vi "Dresden R2R Sputter 03.02.2018 IY24.vi"() -> ()   [LabVIEW 2009] (continued)
        n4396 = Boolean Array To Number(Boolean array=w6390) -> (number=w6389:u32)
        n4397 = Boolean Array To Number(Boolean array=w6370) -> (number=w6369:u32)
        n4398 = Boolean Array To Number(Boolean array=w6382) -> (number=w6383:u32)
        n4399 = Boolean Array To Number(Boolean array=w6357) -> (number=w6358:u32)
        n4400 = Boolean Array To Number(Boolean array=w6346) -> (number=w6345:u32)
        n4401 = Mantissa & Exponent(0:w6389) -> (2:w6388:dbl)  [unwired: 1 out]
        n4402 = Mantissa & Exponent(0:w6369) -> (2:w6366:dbl)  [unwired: 1 out]
        n4403 = Mantissa & Exponent(0:w6383) -> (2:w6378:dbl)  [unwired: 1 out]
        n4404 = Mantissa & Exponent(0:w6358) -> (2:w6361:dbl)  [unwired: 1 out]
        n4405 = Mantissa & Exponent(0:w6345) -> (2:w6344:dbl)  [unwired: 1 out]
        n4406 = case shown="1" w6388 {
          tunnel: [u32[][] [] ("data (RGB format)") w6403 w6404 w6405] -> w6387
          tunnel: w6386 -> [_ w6403 _ _]
          tunnel: w6384 -> [_ _ w6404 _]
          tunnel: w6333 -> [_ _ _ w6405]
          frame #0 {
            (unwired) cluster{"x":i16, "y":i16} {"x"=0, "y"=0} ("top left point(0, 0)")
          }
          frame #1 {
          }
          frame #2 {
          }
          frame #3 {
          }
        }
        n4407 = case shown="1" w6378 {
          tunnel: [u32[][] [] ("data (RGB format)") w6400 w6401] -> w6380
          tunnel: w6379 -> [_ w6400 _]
          tunnel: w6374 -> [_ _ w6401]
          frame #0 {
          }
          frame #1 {
          }
          frame #2 {
          }
        }
        n4408 = case shown="0, Default" w6366 {
          tunnel: w6365 -> [_ w6398]
          tunnel: [u32[][] [] ("data (RGB format)") w6398] -> w6363
          frame #0 {
          }
          frame #1 {
          }
        }
        n4409 = case shown="2" w6361 {
          tunnel: w6356 -> [_ w6395 _]
          tunnel: [u32[][] [] ("data (RGB format)") w6395 w6396] -> w6362
          tunnel: w6355 -> [_ _ w6396]
          frame #0 {
          }
          frame #1 {
          }
          frame #2 {
          }
        }
        n4410 = case shown="0, Default" w6344 {
          tunnel: w6342 -> [_ w6392 _]
          tunnel: [u32[][] [] ("data (RGB format)") w6392 w6393] -> w6343
          tunnel: w6341 -> [_ _ w6393]
          frame #0 {
          }
          frame #1 {
          }
          frame #2 {
          }
        }
        n4411 = call-poly <vilib>:"Draw Unflattened Pixmap.vi"("top left point(0, 0)"=cluster{"x":i16, "y":i16} {"x"=135, "y"=169}, "data (RGB format)"=w6353) -> ("new picture"=w6351:picture)  [unwired: 7 in]
        n4412 = call-poly <vilib>:"Draw Unflattened Pixmap.vi"("picture"=w6351, "top left point(0, 0)"=cluster{"x":i16, "y":i16} {"x"=180, "y"=296}, "data (RGB format)"=w6387) -> ("new picture"=w6381:picture)  [unwired: 6 in]
        n4413 = call-poly <vilib>:"Draw Unflattened Pixmap.vi"("picture"=w6381, "top left point(0, 0)"=cluster{"x":i16, "y":i16} {"x"=563, "y"=309}, "data (RGB format)"=w6380) -> ("new picture"=w6364:picture)  [unwired: 6 in]
        n4414 = call-poly <vilib>:"Draw Unflattened Pixmap.vi"("picture"=w6364, "top left point(0, 0)"=cluster{"x":i16, "y":i16} {"x"=281, "y"=591}, "data (RGB format)"=w6363) -> ("new picture"=w6352:picture)  [unwired: 6 in]
        n4415 = call-poly <vilib>:"Draw Unflattened Pixmap.vi"("picture"=w6352, "top left point(0, 0)"=cluster{"x":i16, "y":i16} {"x"=302, "y"=656}, "data (RGB format)"=w6362) -> ("new picture"=w6347:picture)  [unwired: 6 in]
        n4416 = call-poly <vilib>:"Draw Unflattened Pixmap.vi"("picture"=w6347, "top left point(0, 0)"=cluster{"x":i16, "y":i16} {"x"=487, "y"=251}, "data (RGB format)"=w6343) -> ("new picture"=w6348:picture)  [unwired: 6 in]
      }
      frame #1 {
        # "6"
        # "PET-COOL"
        # "5"
        # "CST-FIX"
        # "4"
        # "CST-FIX"
        # "3"
        # "Magnetron"
        n4417 = property on="Background_ch1_front" class="Pict"() -> ("Mouse"=w6471:T37)  [unwired: 2 in, 2 out]
        n4418 = Unbundle(w6471) -> ("Mouse Position"=w6464:cluster{"X":i32, "Y":i32}, "Mouse Modifiers"=w6472:T38)
        "Mouse Position 2" <- w6464
        n4419 = Unbundle(w6472) -> ("Button Down"=w6430:bool)  [unwired: 3 out]
        n4420 = Unbundle(w6464) -> ("X"=w6408:i32, "Y"=w6407:i32)
        n4421 = In Range and Coerce(upper limit=600, x=w6407, lower limit=320) -> (In Range?=w6465:bool)  [unwired: 1 out]
        n4422 = In Range and Coerce(upper limit=610, x=w6408, lower limit=569) -> (In Range?=w6466:bool)  [unwired: 1 out]
        n4423 = In Range and Coerce(upper limit=525, x=w6408, lower limit=487) -> (In Range?=w6450:bool)  [unwired: 1 out]
        n4424 = In Range and Coerce(upper limit=276, x=w6407, lower limit=257) -> (In Range?=w6451:bool)  [unwired: 1 out]
        n4425 = In Range and Coerce(upper limit=382, x=w6408, lower limit=322) -> (In Range?=w6415:bool)  [unwired: 1 out]
        n4426 = In Range and Coerce(upper limit=333, x=w6407, lower limit=172) -> (In Range?=w6416:bool)  [unwired: 1 out]
        n4427 = In Range and Coerce(upper limit=473, x=w6408, lower limit=435) -> (In Range?=w6418:bool)  [unwired: 1 out]
        n4428 = In Range and Coerce(upper limit=324, x=w6407, lower limit=204) -> (In Range?=w6417:bool)  [unwired: 1 out]
        n4429 = In Range and Coerce(upper limit=367, x=w6408, lower limit=247) -> (In Range?=w6429:bool)  [unwired: 1 out]
        n4430 = In Range and Coerce(upper limit=680, x=w6407, lower limit=637) -> (In Range?=w6440:bool)  [unwired: 1 out]
        n4431 = In Range and Coerce(upper limit=273, x=w6408, lower limit=234) -> (In Range?=w6420:bool)  [unwired: 1 out]
        n4432 = In Range and Coerce(upper limit=324, x=w6407, lower limit=204) -> (In Range?=w6419:bool)  [unwired: 1 out]
        n4433 = And(x=w6420, y=w6419) -> (x .and. y?=w6410:bool)
        n4434 = And(x=w6415, y=w6416) -> (x .and. y?=w6406:bool)
        n4435 = And(x=w6418, y=w6417) -> (x .and. y?=w6409:bool)
        n4436 = And(x=w6466, y=w6465) -> (x .and. y?=w6454:bool)
        n4437 = And(x=w6450, y=w6451) -> (x .and. y?=w6445:bool)
        n4438 = And(x=w6429, y=w6440) -> (x .and. y?=w6439:bool)
        n4439 = And(x=w6430, y=w6454) -> (x .and. y?=w6432:bool)
        n4440 = And(x=w6430, y=w6445) -> (x .and. y?=w6431:bool)
        n4441 = case shown="True" w6432 {
          frame #0 {
          }
          frame #1 {
            "Gv_timer_front_ch4_3" <- TRUE ("Gv_timer_front_ch1_2")
          }
        }
        n4442 = case shown="True" w6431 {
          frame #0 {
          }
          frame #1 {
            "Trns_gv_bp_ch4_front" <- TRUE ("Gv_timer_front_ch1_2")
          }
        }
        n4443 = local read "Gv_timer_front_ch4_3"() -> (w6434:bool)
        n4444 = local read "Trns_gv_bp_ch4_front"() -> (w6433:bool)
        n4445 = Build Array(FALSE ("element"), w6454, w6445, w6439, w6410, w6409, w6406) -> (w6453:bool[])
        n4446 = Boolean Array To Number(Boolean array=w6453) -> (number=w6462:u32)
        n4447 = feedback #122() -> (w6436:bool)  [unwired: 1 in]
        n4448 = Mantissa & Exponent(0:w6462) -> (2:w6457:dbl)  [unwired: 1 out]
        n4449 = feedback #123() -> (w6437:bool)  [unwired: 1 in]
        n4450 = case shown="True" w6433 {
          tunnel: [TRUE FALSE] -> w6435
          tunnel: w6436 -> [_ w6481]
          frame #0 {
          }
          frame #1 {
            n4451 = call "Elapsed Time49"("Reset"=w6481) -> ("Elapsed Time (s)"=w6478:dbl)  [unwired: 11 in, 7 out]
            n4452 = Greater?(x=w6478, y=3.0) -> (0:w6479:bool)
            n4453 = In Range and Coerce(upper limit=3.0, x=w6478, lower limit=0.0) -> (In Range?=w6474:bool)  [unwired: 1 out]
            n4454 = Not(x=w6479) -> (.not. x?=w6475:bool)
            n4455 = local write "Trns_gv_bp_ch4_front"(w6475) -> ()
            n4456 = property on="Ch4_Trns_gv_bp_front_gui" class="TabCtl (strict)"("Visible"=w6474) -> ()  [unwired: 2 in, 2 out]
          }
        }
        n4457 = case shown="True" w6434 {
          tunnel: [TRUE FALSE] -> w6438
          tunnel: w6437 -> [_ w6491]
          frame #0 {
          }
          frame #1 {
            n4458 = call "Elapsed Time48"("Reset"=w6491) -> ("Elapsed Time (s)"=w6488:dbl)  [unwired: 11 in, 7 out]
            n4459 = Greater?(x=w6488, y=3.0) -> (0:w6489:bool)
            n4460 = In Range and Coerce(upper limit=3.0, x=w6488, lower limit=0.0) -> (In Range?=w6484:bool)  [unwired: 1 out]
            n4461 = Not(x=w6489) -> (.not. x?=w6485:bool)
            n4462 = property on="Ch3_4_Gv_timer_front_gui" class="TabCtl (strict)"("Visible"=w6484) -> ()  [unwired: 2 in, 2 out]
            n4463 = local write "Gv_timer_front_ch4_3"(w6485) -> ()
          }
        }
        n4464 = case shown="2" w6457 {
          tunnel: ["" ("text") "GV" ("text") "GV-BP" ("text") "MG" ("text") "CST-FIX" ("text") "CST-FIX" ("text") "PET-COOL" ("text")] -> w6459
          tunnel: ["" ("DESCRIPTION") "Gate Valve" ("DESCRIPTION") "Gate Valve-By Pass" ("DESCRIPTION") "Magnetron" ("DESCRIPTION") "Casette Fix" ("DESCRIPTION") "Casette Fix" ("DESCRIPTION") "Petfolio Cool" ("DESCRIPTION")] -> w6458
          tunnel: [cluster{"x":i16, "y":i16} {"x"=0, "y"=0} ("origin") cluster{"x":i16, "y":i16} {"x"=629, "y"=455} ("origin") cluster{"x":i16, "y":i16} {"x"=504, "y"=231} ("origin") cluster{"x":i16, "y":i16} {"x"=338, "y"=709} ("origin") cluster{"x":i16, "y":i16} {"x"=225, "y"=176} ("origin") cluster{"x":i16, "y":i16} {"x"=426, "y"=176} ("origin") cluster{"x":i16, "y":i16} {"x"=315, "y"=144} ("origin")] -> w6456
          frame #0 {
          }
          frame #1 {
          }
          frame #2 {
          }
          frame #3 {
          }
          frame #4 {
          }
          frame #5 {
          }
          frame #6 {
          }
        }
        n4465 = local write "DESCRIPTION"(w6458) -> ()
        n4466 = call <vilib>:"Draw Text at Point.vi"("[user-specified font]"=T35 {"Font Name:"="BOLD\n", "Size"=18, "Strikeout?"=FALSE, "Italic?"=FALSE, "Underline?"=FALSE, "Outline?"=FALSE, "Shadow?"=FALSE, "Bold?"=TRUE} ("[user-specified font] 2"), "desired font(Application)"=T36."User-specified Font", "text"=w6459, "origin"=w6456, "picture"=w6461) -> ("new picture"=w6460:picture)  [unwired: 5 in, 1 out]
      }
      frame #2 {
        n4467 = disable-structure shown="Disabled" {
          frame #0 {
            n4468 = stacked-sequence {
              frame #0 {
                n4469 = Read from Text File(file (use dialog)=path path "") -> (text=→"Chamber2":string)  [unwired: 3 in, 3 out]
                n4470 = Read from Text File(file (use dialog)=path path "") -> (text=→"Chamber3":string)  [unwired: 3 in, 3 out]
                n4471 = Read from Text File(file (use dialog)=path path "") -> (text=→"Chamber4":string)  [unwired: 3 in, 3 out]
                n4472 = Read from Text File(file (use dialog)=path path "") -> (text=→"Substrate":string)  [unwired: 3 in, 3 out]
              }
            }
          }
          frame #1 {
          }
        }
      }
    }
    "Background_ch1_front" <- w5967
    n4473 = stacked-sequence {
      tunnel: w5981 -> [w6085 _]
      tunnel: [_ w6220] -> w5966
      tunnel: w5971 -> [w6080 _]
      tunnel: w5970 -> [w6079 _]
      tunnel: w5969 -> [w6067 _]
      tunnel: w5968 -> [w6066 _]
      tunnel: w5962 -> [w6063 _]
      tunnel: w5963 -> [w6064 _]
      tunnel: w5961 -> [w6047 _]
      tunnel: w5960 -> [w6046 _]
      tunnel: w5958 -> [w6043 _]
      tunnel: w5959 -> [w6044 _]
      tunnel: w5956 -> [w6033 _]
      tunnel: w5957 -> [w6034 _]
      tunnel: w5952 -> [w6007 _]
      tunnel: w5955 -> [w6018 _]
      tunnel: w5954 -> [w6010 _]
      tunnel: w5953 -> [w6009 _]
      tunnel: w5951 -> [w5999 _]
      tunnel: w5950 -> [w5998 _]
      frame #0 {
        n4474 = Build Array(FALSE ("element"), "ch4_atm_fail_top", "ch4_atm_on_top") -> (w6059:bool[])
        n4475 = Build Array(FALSE ("element"), "ch4_pg_fail_top", "ch4_pg_on_top") -> (w6051:bool[])
        n4476 = Build Array(FALSE ("element"), "ch4_cc_fail_top", "ch4_cc_on_top") -> (w6039:bool[])
        n4477 = Build Array(FALSE ("element"), "ch4_bg_fail_top", "ch4_bg_on_top") -> (w6029:bool[])
        n4478 = Build Array(FALSE ("element"), "gv top open ch_4_3", "gv top failed ch4_3") -> (w6072:bool[])
        n4479 = Build Array(FALSE ("element"), "chamber 4 top piston open", "chamber 4 top piston failed") -> (w6084:bool[])
        n4480 = Build Array(FALSE ("element"), "ch4_bg_bv_fail_top", "ch4_bg_bv_on_top") -> (w6022:bool[])
        n4481 = Build Array(FALSE ("element"), "ch4_sov_Ar_on_top", "ch4_sov_Ar_fail_top") -> (w6003:bool[])
        n4482 = Build Array(FALSE ("element"), "Trns_gv_bp_ch4_on_top", "Trns_gv_bp_ch4_fail_top") -> (w6014:bool[])
        n4483 = Boolean Array To Number(Boolean array=w6059) -> (number=w6058:u32)
        n4484 = Boolean Array To Number(Boolean array=w6051) -> (number=w6052:u32)
        n4485 = Boolean Array To Number(Boolean array=w6039) -> (number=w6038:u32)
        n4486 = Boolean Array To Number(Boolean array=w6029) -> (number=w6028:u32)
        n4487 = Boolean Array To Number(Boolean array=w6072) -> (number=w6073:u32)
        n4488 = Boolean Array To Number(Boolean array=w6084) -> (number=w6083:u32)
        n4489 = Boolean Array To Number(Boolean array=w6022) -> (number=w6023:u32)
        n4490 = Boolean Array To Number(Boolean array=w6003) -> (number=w6004:u32)
        n4491 = Boolean Array To Number(Boolean array=w6014) -> (number=w6013:u32)
        n4492 = Mantissa & Exponent(0:w6058) -> (2:w6057:dbl)  [unwired: 1 out]
        n4493 = Mantissa & Exponent(0:w6052) -> (2:w6053:dbl)  [unwired: 1 out]
        n4494 = Mantissa & Exponent(0:w6038) -> (2:w6037:dbl)  [unwired: 1 out]
        n4495 = Mantissa & Exponent(0:w6028) -> (2:w6027:dbl)  [unwired: 1 out]
        n4496 = Mantissa & Exponent(0:w6073) -> (2:w6074:dbl)  [unwired: 1 out]
        n4497 = Mantissa & Exponent(0:w6083) -> (2:w6082:dbl)  [unwired: 1 out]
        n4498 = Mantissa & Exponent(0:w6023) -> (2:w6024:dbl)  [unwired: 1 out]
        n4499 = Mantissa & Exponent(0:w6004) -> (2:w6005:dbl)  [unwired: 1 out]
        n4500 = Mantissa & Exponent(0:w6013) -> (2:w6012:dbl)  [unwired: 1 out]
        n4501 = case shown="0, Default" w6057 {
          tunnel: w6064 -> [_ w6105 _]
          tunnel: [u32[][] [] ("data (RGB format)") w6105 w6106] -> w6056
          tunnel: w6063 -> [_ _ w6106]
          frame #0 {
          }
          frame #1 {
          }
          frame #2 {
          }
        }
        n4502 = case shown="0, Default" w6053 {
          tunnel: w6046 -> [_ w6102 _]
          tunnel: [u32[][] [] ("data (RGB format)") w6102 w6103] -> w6054
          tunnel: w6047 -> [_ _ w6103]
          frame #0 {
          }
          frame #1 {
          }
          frame #2 {
          }
        }
        n4503 = case shown="1" w6037 {
          tunnel: w6044 -> [_ w6099 _]
          tunnel: [u32[][] [] ("data (RGB format)") w6099 w6100] -> w6036
          tunnel: w6043 -> [_ _ w6100]
          frame #0 {
          }
          frame #1 {
          }
          frame #2 {
          }
        }
        n4504 = case shown="0, Default" w6027 {
          tunnel: w6034 -> [_ w6096 _]
          tunnel: [u32[][] [] ("data (RGB format)") w6096 w6097] -> w6026
          tunnel: w6033 -> [_ _ w6097]
          frame #0 {
          }
          frame #1 {
          }
          frame #2 {
          }
        }
        n4505 = case shown="2" w6074 {
          tunnel: w6066 -> [_ w6110 _]
          tunnel: [u32[][] [] ("data (RGB format)") w6110 w6112] -> w6075
          tunnel: w6067 -> [_ _ w6112]
          tunnel: [cluster{"x":i16, "y":i16} {"x"=0, "y"=0} ("top left point(0, 0)") cluster{"x":i16, "y":i16} {"x"=521, "y"=342} ("top left point(0, 0)") cluster{"x":i16, "y":i16} {"x"=524, "y"=342} ("top left point(0, 0)")] -> w5985
          frame #0 {
          }
          frame #1 {
          }
          frame #2 {
          }
        }
        n4506 = case shown="1" w6082 {
          tunnel: w6079 -> [_ w6116 _]
          tunnel: [u32[][] [] ("data (RGB format)") w6116 w6118] -> w6081
          tunnel: w6080 -> [_ _ w6118]
          tunnel: [cluster{"x":i16, "y":i16} {"x"=0, "y"=0} ("top left point(0, 0)") cluster{"x":i16, "y":i16} {"x"=103, "y"=167} ("top left point(0, 0)") cluster{"x":i16, "y":i16} {"x"=100, "y"=167} ("top left point(0, 0)")] -> w5994
          frame #0 {
          }
          frame #1 {
          }
          frame #2 {
          }
        }
        n4507 = case shown="0, Default" w6024 {
          tunnel: w6018 -> [_ _ w6094]
          tunnel: w6007 -> [_ w6093 _]
          tunnel: [u32[][] [] ("data (RGB format)") w6093 w6094] -> w5989
          frame #0 {
          }
          frame #1 {
          }
          frame #2 {
          }
        }
        n4508 = case shown="1" w6005 {
          tunnel: w5999 -> [_ w6087 _]
          tunnel: [u32[][] [] ("data (RGB format)") w6087 w6088] -> w6006
          tunnel: w5998 -> [_ _ w6088]
          frame #0 {
          }
          frame #1 {
          }
          frame #2 {
          }
        }
        n4509 = case shown="0, Default" w6012 {
          tunnel: w6010 -> [_ w6090 _]
          tunnel: [u32[][] [] ("data (RGB format)") w6090 w6091] -> w6011
          tunnel: w6009 -> [_ _ w6091]
          frame #0 {
          }
          frame #1 {
          }
          frame #2 {
          }
        }
        n4510 = call-poly <vilib>:"Draw Unflattened Pixmap.vi"("top left point(0, 0)"=cluster{"x":i16, "y":i16} {"x"=100, "y"=167}, "data (RGB format)"=w6085) -> ("new picture"=w6065:picture)  [unwired: 7 in]
        n4511 = call-poly <vilib>:"Draw Unflattened Pixmap.vi"("picture"=w6065, "top left point(0, 0)"=w5994, "data (RGB format)"=w6081) -> ("new picture"=w6071:picture)  [unwired: 6 in]
        n4512 = call-poly <vilib>:"Draw Unflattened Pixmap.vi"("picture"=w6071, "top left point(0, 0)"=w5985, "data (RGB format)"=w6075) -> ("new picture"=w6055:picture)  [unwired: 6 in]
        n4513 = call-poly <vilib>:"Draw Unflattened Pixmap.vi"("picture"=w6055, "top left point(0, 0)"=cluster{"x":i16, "y":i16} {"x"=434, "y"=639} ("top left point(0, 0) 3"), "data (RGB format)"=w6056) -> ("new picture"=w6045:picture)  [unwired: 6 in]
        n4514 = call-poly <vilib>:"Draw Unflattened Pixmap.vi"("picture"=w6045, "top left point(0, 0)"=cluster{"x":i16, "y":i16} {"x"=154, "y"=618} ("top left point(0, 0) 4"), "data (RGB format)"=w6054) -> ("new picture"=w6035:picture)  [unwired: 6 in]
        n4515 = call-poly <vilib>:"Draw Unflattened Pixmap.vi"("picture"=w6035, "top left point(0, 0)"=cluster{"x":i16, "y":i16} {"x"=228, "y"=625} ("top left point(0, 0) 3"), "data (RGB format)"=w6036) -> ("new picture"=w6025:picture)  [unwired: 6 in]
        n4516 = call-poly <vilib>:"Draw Unflattened Pixmap.vi"("picture"=w6025, "top left point(0, 0)"=cluster{"x":i16, "y":i16} {"x"=331, "y"=673} ("top left point(0, 0) 3"), "data (RGB format)"=w6026) -> ("new picture"=w6017:picture)  [unwired: 6 in]
        n4517 = call-poly <vilib>:"Draw Unflattened Pixmap.vi"("picture"=w6017, "top left point(0, 0)"=cluster{"x":i16, "y":i16} {"x"=319, "y"=636} ("top left point(0, 0) 3"), "data (RGB format)"=w5989) -> ("new picture"=w6008:picture)  [unwired: 6 in]
        n4518 = call-poly <vilib>:"Draw Unflattened Pixmap.vi"("picture"=w6008, "top left point(0, 0)"=cluster{"x":i16, "y":i16} {"x"=444, "y"=283} ("top left point(0, 0) 3"), "data (RGB format)"=w6011) -> ("new picture"=w5997:picture)  [unwired: 6 in]
        n4519 = call-poly <vilib>:"Draw Unflattened Pixmap.vi"("picture"=w5997, "top left point(0, 0)"="top left point(0, 0) 3", "data (RGB format)"=w6006) -> ("new picture"=w5996:picture)  [unwired: 6 in]
      }
      frame #1 {
        # "12"
        # "MFC"
        # "11"
        # "PET-COOL"
        # "10"
        # "CST-FIX"
        # "9"
        # "CST-FIX"
        n4520 = property on="Background_ch1_top" class="Pict"() -> ("Mouse"=w6226:T37)  [unwired: 2 in, 2 out]
        n4521 = Unbundle(w6226) -> ("Mouse Position"=w6225:cluster{"X":i32, "Y":i32}, "Mouse Modifiers"=w6227:T38)
        "Mouse Position 3" <- w6225
        n4522 = Unbundle(w6227) -> ("Button Down"=w6167:bool)  [unwired: 3 out]
        n4523 = Unbundle(w6225) -> ("X"=w6121:i32, "Y"=w6120:i32)
        n4524 = In Range and Coerce(upper limit=599, x=w6120, lower limit=354) -> (In Range?=w6233:bool)  [unwired: 1 out]
        n4525 = In Range and Coerce(upper limit=564, x=w6121, lower limit=528) -> (In Range?=w6232:bool)  [unwired: 1 out]
        n4526 = In Range and Coerce(upper limit=676, x=w6120, lower limit=645) -> (In Range?=w6234:bool)  [unwired: 1 out]
        n4527 = In Range and Coerce(upper limit=543, x=w6121, lower limit=513) -> (In Range?=w6123:bool)  [unwired: 1 out]
        n4528 = In Range and Coerce(upper limit=244, x=w6120, lower limit=196) -> (In Range?=w6122:bool)  [unwired: 1 out]
        n4529 = In Range and Coerce(upper limit=652, x=w6120, lower limit=627) -> (In Range?=w6212:bool)  [unwired: 1 out]
        n4530 = In Range and Coerce(upper limit=335, x=w6121, lower limit=281) -> (In Range?=w6136:bool)  [unwired: 1 out]
        n4531 = In Range and Coerce(upper limit=391, x=w6120, lower limit=168) -> (In Range?=w6137:bool)  [unwired: 1 out]
        n4532 = In Range and Coerce(upper limit=479, x=w6121, lower limit=436) -> (In Range?=w6235:bool)  [unwired: 1 out]
        n4533 = In Range and Coerce(upper limit=180, x=w6121, lower limit=154) -> (In Range?=w6211:bool)  [unwired: 1 out]
        n4534 = In Range and Coerce(upper limit=411, x=w6121, lower limit=359) -> (In Range?=w6139:bool)  [unwired: 1 out]
        n4535 = In Range and Coerce(upper limit=367, x=w6120, lower limit=215) -> (In Range?=w6138:bool)  [unwired: 1 out]
        n4536 = In Range and Coerce(upper limit=669, x=w6120, lower limit=636) -> (In Range?=w6201:bool)  [unwired: 1 out]
        n4537 = In Range and Coerce(upper limit=661, x=w6120, lower limit=636) -> (In Range?=w6185:bool)  [unwired: 1 out]
        n4538 = In Range and Coerce(upper limit=257, x=w6121, lower limit=206) -> (In Range?=w6141:bool)  [unwired: 1 out]
        n4539 = In Range and Coerce(upper limit=367, x=w6120, lower limit=215) -> (In Range?=w6140:bool)  [unwired: 1 out]
        n4540 = In Range and Coerce(upper limit=266, x=w6121, lower limit=228) -> (In Range?=w6202:bool)  [unwired: 1 out]
        n4541 = In Range and Coerce(upper limit=355, x=w6121, lower limit=321) -> (In Range?=w6186:bool)  [unwired: 1 out]
        n4542 = In Range and Coerce(upper limit=310, x=w6120, lower limit=286) -> (In Range?=w6182:bool)  [unwired: 1 out]
        n4543 = In Range and Coerce(upper limit=708, x=w6120, lower limit=683) -> (In Range?=w6197:bool)  [unwired: 1 out]
        n4544 = In Range and Coerce(upper limit=482, x=w6121, lower limit=445) -> (In Range?=w6181:bool)  [unwired: 1 out]
        n4545 = In Range and Coerce(upper limit=357, x=w6121, lower limit=330) -> (In Range?=w6196:bool)  [unwired: 1 out]
        n4546 = In Range and Coerce(upper limit=254, x=w6120, lower limit=204) -> (In Range?=w6171:bool)  [unwired: 1 out]
        n4547 = In Range and Coerce(upper limit=484, x=w6121, lower limit=464) -> (In Range?=w6172:bool)  [unwired: 1 out]
        n4548 = And(x=w6141, y=w6140) -> (x .and. y?=w6131:bool)
        n4549 = And(x=w6123, y=w6122) -> (x .and. y?=w6119:bool)
        n4550 = And(x=w6136, y=w6137) -> (x .and. y?=w6129:bool)
        n4551 = And(x=w6139, y=w6138) -> (x .and. y?=w6130:bool)
        n4552 = And(x=w6232, y=w6233) -> (x .and. y?=w6214:bool)
        n4553 = And(x=w6235, y=w6234) -> (x .and. y?=w6213:bool)
        n4554 = And(x=w6211, y=w6212) -> (x .and. y?=w6199:bool)
        n4555 = And(x=w6202, y=w6201) -> (x .and. y?=w6198:bool)
        n4556 = And(x=w6186, y=w6185) -> (x .and. y?=w6169:bool)
        n4557 = And(x=w6181, y=w6182) -> (x .and. y?=w6166:bool)
        n4558 = And(x=w6196, y=w6197) -> (x .and. y?=w6191:bool)
        n4559 = And(x=w6172, y=w6171) -> (x .and. y?=w6168:bool)
        n4560 = And(x=w6167, y=w6214) -> (x .and. y?=w6215:bool)
        n4561 = And(x=w6167, y=w6198) -> (x .and. y?=w6200:bool)
        n4562 = And(x=w6167, y=w6169) -> (x .and. y?=w6184:bool)
        n4563 = And(x=w6167, y=w6166) -> (x .and. y?=w6183:bool)
        n4564 = And(x=w6167, y=w6168) -> (x .and. y?=w6170:bool)
        n4565 = case shown="True" w6215 {
          frame #0 {
          }
          frame #1 {
            "Gv_timer_top_ch3_4" <- TRUE ("Gv_timer_top_ch1_2")
          }
        }
        n4566 = case shown="True" w6200 {
          frame #0 {
          }
          frame #1 {
            "ch4_cc_timer_top" <- TRUE ("ch1_atm_timer_top")
          }
        }
        n4567 = case shown="True" w6184 {
          frame #0 {
          }
          frame #1 {
            "ch4_bg_bv_timer_top" <- TRUE ("ch1_atm_timer_top")
          }
        }
        n4568 = case shown="True" w6183 {
          frame #0 {
          }
          frame #1 {
            "ch4_bv_timer_top" <- TRUE ("ch1_atm_timer_top")
          }
        }
        n4569 = case shown="True" w6170 {
          frame #0 {
          }
          frame #1 {
            "ch4_sov_Ar_timer_top" <- TRUE ("ch1_atm_timer_top")
          }
        }
        n4570 = Build Array(FALSE ("element"), w6214, w6213, w6199, w6198, w6191, w6169, w6166, w6168, w6131, w6130, w6129, w6119) -> (w6224:bool[])
        n4571 = Boolean Array To Number(Boolean array=w6224) -> (number=w6223:u32)
        n4572 = local read "ch4_bv_timer_top"() -> (w6151:bool)
        n4573 = local read "ch4_bg_bv_timer_top"() -> (w6152:bool)
        n4574 = local read "ch4_sov_Ar_timer_top"() -> (w6150:bool)
        n4575 = local read "Gv_timer_top_ch3_4"() -> (w6154:bool)
        n4576 = local read "ch4_cc_timer_top"() -> (w6153:bool)
        n4577 = Mantissa & Exponent(0:w6223) -> (2:w6221:dbl)  [unwired: 1 out]
        n4578 = case shown="6" w6221 {
          tunnel: ["" ("text") "GV" ("text") "CH-ATM" ("text") "CH-PG" ("text") "CH-CC" ("text") "CH-BG" ("text") "BG-BV" ("text") "GV-BP" ("text") "SOV-Ar" ("text") "CST-FIX" ("text") "CST-FIX" ("text") "PET-COOL" ("text") "MFC" ("text")] -> w6217
          tunnel: ["" ("DESCRIPTION") "Gate Valve" ("DESCRIPTION") "Chamber-Atmospheric Switch" ("DESCRIPTION") "Chamber - Pirani Gauge" ("DESCRIPTION") "Chamber-Cold Cathode" ("DESCRIPTION") "Chamber-Baratron Gauge" ("DESCRIPTION") "Baratron Gauge- Block Valve" ("DESCRIPTION") "Gate Valve-By Pass" ("DESCRIPTION") "Shut Off Valve-Ar Gas" ("DESCRIPTION") "Casette Fix" ("DESCRIPTION") "Casette Fix" ("DESCRIPTION") "Petfolio Cool" ("DESCRIPTION") "Mass Flow Control" ("DESCRIPTION")] -> w6216
          tunnel: [cluster{"x":i16, "y":i16} {"x"=0, "y"=0} ("origin") cluster{"x":i16, "y":i16} {"x"=587, "y"=463} ("origin") cluster{"x":i16, "y":i16} {"x"=457, "y"=689} ("origin") cluster{"x":i16, "y":i16} {"x"=140, "y"=663} ("origin") cluster{"x":i16, "y":i16} {"x"=227, "y"=679} ("origin") cluster{"x":i16, "y":i16} {"x"=321, "y"=712} ("origin") cluster{"x":i16, "y":i16} {"x"=367, "y"=641} ("origin") cluster{"x":i16, "y":i16} {"x"=438, "y"=269} ("origin") cluster{"x":i16, "y":i16} {"x"=455, "y"=186} ("origin") cluster{"x":i16, "y":i16} {"x"=192, "y"=167} ("origin") cluster{"x":i16, "y":i16} {"x"=359, "y"=167} ("origin") cluster{"x":i16, "y":i16} {"x"=270, "y"=139} ("origin") cluster{"x":i16, "y":i16} {"x"=512, "y"=180} ("origin")] -> w6128
          frame #0 {
          }
          frame #1 {
          }
          frame #2 {
          }
          frame #3 {
          }
          frame #4 {
          }
          frame #5 {
          }
          frame #6 {
          }
          frame #7 {
          }
          frame #8 {
          }
          frame #9 {
          }
          frame #10 {
          }
          frame #11 {
          }
          frame #12 {
          }
        }
        n4579 = feedback #124() -> (w6158:bool)  [unwired: 1 in]
        n4580 = feedback #125() -> (w6163:bool)  [unwired: 1 in]
        n4581 = feedback #126() -> (w6162:bool)  [unwired: 1 in]
        n4582 = feedback #127() -> (w6159:bool)  [unwired: 1 in]
        n4583 = feedback #128() -> (w6155:bool)  [unwired: 1 in]
        n4584 = case shown="True" w6151 {
          tunnel: [TRUE FALSE] -> w6157
          tunnel: w6158 -> [_ w6258]
          frame #0 {
          }
          frame #1 {
            n4585 = call "Elapsed Time53"("Reset"=w6258) -> ("Elapsed Time (s)"=w6255:dbl)  [unwired: 11 in, 7 out]
            n4586 = Greater?(x=w6255, y=3.0) -> (0:w6256:bool)
            n4587 = In Range and Coerce(upper limit=3.0, x=w6255, lower limit=0.0) -> (In Range?=w6251:bool)  [unwired: 1 out]
            n4588 = Not(x=w6256) -> (.not. x?=w6252:bool)
            n4589 = local write "ch4_bv_timer_top"(w6252) -> ()
            n4590 = property on="Ch4_Trns_gv_bp_timer_top__gui" class="TabCtl (strict)"("Visible"=w6251) -> ()  [unwired: 2 in, 2 out]
          }
        }
        n4591 = case shown="True" w6154 {
          tunnel: [TRUE FALSE] -> w6164
          tunnel: w6163 -> [_ w6287]
          frame #0 {
          }
          frame #1 {
            n4592 = call "Elapsed Time50"("Reset"=w6287) -> ("Elapsed Time (s)"=w6285:dbl)  [unwired: 11 in, 7 out]
            n4593 = Greater?(x=w6285, y=3.0) -> (0:w6282:bool)
            n4594 = In Range and Coerce(upper limit=3.0, x=w6285, lower limit=0.0) -> (In Range?=w6281:bool)  [unwired: 1 out]
            n4595 = Not(x=w6282) -> ()  [unwired: 1 out]
            n4596 = property on="Gv_ch4_3_timer_top_gui" class="TabCtl (strict)"("Visible"=w6281) -> ()  [unwired: 2 in, 2 out]
            n4597 = local write "Gv_timer_top_ch3_4"(w6282) -> ()
          }
        }
        n4598 = case shown="True" w6153 {
          tunnel: [TRUE FALSE] -> w6161
          tunnel: w6162 -> [_ w6278]
          frame #0 {
          }
          frame #1 {
            n4599 = call "Elapsed Time51"("Reset"=w6278) -> ("Elapsed Time (s)"=w6275:dbl)  [unwired: 11 in, 7 out]
            n4600 = Greater?(x=w6275, y=3.0) -> (0:w6276:bool)
            n4601 = In Range and Coerce(upper limit=3.0, x=w6275, lower limit=0.0) -> (In Range?=w6271:bool)  [unwired: 1 out]
            n4602 = Not(x=w6276) -> (.not. x?=w6272:bool)
            n4603 = local write "ch4_cc_timer_top"(w6272) -> ()
            n4604 = property on="Ch4_Cc_timer_top__gui" class="TabCtl (strict)"("Visible"=w6271) -> ()  [unwired: 2 in, 2 out]
          }
        }
        n4605 = case shown="True" w6152 {
          tunnel: [TRUE FALSE] -> w6160
          tunnel: w6159 -> [_ w6268]
          frame #0 {
          }
          frame #1 {
            n4606 = call "Elapsed Time52"("Reset"=w6268) -> ("Elapsed Time (s)"=w6265:dbl)  [unwired: 11 in, 7 out]
            n4607 = Greater?(x=w6265, y=3.0) -> (0:w6266:bool)
            n4608 = In Range and Coerce(upper limit=3.0, x=w6265, lower limit=0.0) -> (In Range?=w6261:bool)  [unwired: 1 out]
            n4609 = Not(x=w6266) -> (.not. x?=w6262:bool)
            n4610 = local write "ch4_bg_bv_timer_top"(w6262) -> ()
            n4611 = property on="Ch4_Bg_bv_timer_top__gui" class="TabCtl (strict)"("Visible"=w6261) -> ()  [unwired: 2 in, 2 out]
          }
        }
        n4612 = case shown="True" w6150 {
          tunnel: [TRUE FALSE] -> w6156
          tunnel: w6155 -> [_ w6248]
          frame #0 {
          }
          frame #1 {
            n4613 = call "Elapsed Time54"("Reset"=w6248) -> ("Elapsed Time (s)"=w6245:dbl)  [unwired: 11 in, 7 out]
            n4614 = Greater?(x=w6245, y=3.0) -> (0:w6246:bool)
            n4615 = In Range and Coerce(upper limit=3.0, x=w6245, lower limit=0.0) -> (In Range?=w6241:bool)  [unwired: 1 out]
            n4616 = Not(x=w6246) -> (.not. x?=w6242:bool)
            n4617 = local write "ch4_sov_Ar_timer_top"(w6242) -> ()
            n4618 = property on="Ch4_Sov_Ar_timer_top__gui" class="TabCtl (strict)"("Visible"=w6241) -> ()  [unwired: 2 in, 2 out]
          }
        }
        n4619 = local write "DESCRIPTION"(w6216) -> ()
        n4620 = call <vilib>:"Draw Text at Point.vi"("[user-specified font]"=T35 {"Font Name:"="BOLD", "Size"=18, "Strikeout?"=FALSE, "Italic?"=FALSE, "Underline?"=FALSE, "Outline?"=FALSE, "Shadow?"=FALSE, "Bold?"=TRUE} ("[user-specified font] 3"), "desired font(Application)"=T36."User-specified Font", "text"=w6217, "origin"=w6128, "picture"=w6219) -> ("new picture"=w6220:picture)  [unwired: 5 in, 1 out]
      }
    }
    "Background_ch1_top" <- w5966
    n4621 = Wait Until Next ms Multiple(millisecond multiple=u32 100) -> ()  [unwired: 1 out]
  }
  n4622 = while {
    tunnel: w571 -> [w6564]
    tunnel: w570 -> [w6563]
    tunnel: w569 -> [w6562]
    tunnel: w566 -> [w6559]
    tunnel: w567 -> [w6560]
    tunnel: w568 -> [w6561]
    tunnel: w565 -> [w6558]
    tunnel: w564 -> [w6557]
    tunnel: w563 -> [w6556]
    tunnel: w562 -> [w6555]
    tunnel: w561 -> [w6554]
    tunnel: w560 -> [w6553]
    tunnel: w559 -> [w6552]
    tunnel: w558 -> [w6551]
    tunnel: w354 -> [w6548]
    tunnel: w353 -> [w6547]
    tunnel: w291 -> [w6546]
    tunnel: w290 -> [w6545]
    tunnel: w245 -> [w6544]
    tunnel: w244 -> [w6543]
    tunnel: w243 -> [w6542]
    tunnel: w242 -> [w6541]
    tunnel: w241 -> [w6540]
    tunnel: w240 -> [w6539]
    tunnel: w239 -> [w6538]
    tunnel: w238 -> [w6537]
    tunnel: w237 -> [w6536]
    tunnel: w236 -> [w6535]
    tunnel: w235 -> [w6534]
    tunnel: w234 -> [w6533]
    tunnel: w233 -> [w6532]
    tunnel: w232 -> [w6531]
    tunnel: w152 -> [w6530]
    tunnel: w151 -> [w6529]
    tunnel: w144 -> [w6528]
    tunnel: w143 -> [w6527]
    tunnel: w138 -> [w6526]
    tunnel: w137 -> [w6525]
    stop <- FALSE stop-if-true
    n4623 = stacked-sequence {
      tunnel: w6564 -> [w7066 _]
      tunnel: w6563 -> [w7065 _]
      tunnel: w6562 -> [w7064 _]
      tunnel: [_ w7167] -> w6550
      tunnel: w6558 -> [w7063 _]
      tunnel: w6557 -> [w7043 _]
      tunnel: w6556 -> [w7042 _]
      tunnel: w6555 -> [w7040 _]
      tunnel: w6554 -> [w7038 _]
      tunnel: w6553 -> [w7039 _]
      tunnel: w6548 -> [w7023 _]
      tunnel: w6547 -> [w7022 _]
      tunnel: w6528 -> [w7007 _]
      tunnel: w6527 -> [w7006 _]
      tunnel: w6526 -> [w6999 _]
      tunnel: w6525 -> [w6994 _]
      frame #0 {
        n4624 = Build Array(FALSE ("element"), "magnetron on_ch3") -> (w7048:bool[])
        n4625 = Build Array(FALSE ("element"), "chamber3 front piston open drum failed", "chamber3 front piston failed drum open", "chamber3 front piston open") -> (w7067:bool[])
        n4626 = Build Array(FALSE ("element"), "gv front_open_ch3_4", "gv front failed_ch3_4") -> (w7045:bool[])
        n4627 = Build Array(FALSE ("element"), "magnetron water cooled on_ch3", "magnetron water cooled failed_ch3") -> (w7056:bool[])
        n4628 = Build Array(FALSE ("element"), "Ch3_trns_gv_bp2_on_front", "Ch3_trns_gv_bp2_fail_front") -> (w7005:bool[])
        n4629 = Build Array(FALSE ("element"), "gv front failed_ch3_2", "gv front open_ch3_2") -> (w7029:bool[])
        n4630 = Build Array(FALSE ("element"), "Ch3_trns_gv_bp_fail_front", "Ch3_trns_gv_bp_on_front") -> (w7008:bool[])
        n4631 = Boolean Array To Number(Boolean array=w7048) -> (number=w7049:u32)
        n4632 = Boolean Array To Number(Boolean array=w7067) -> (number=w7068:u32)
        n4633 = Boolean Array To Number(Boolean array=w7045) -> (number=w7044:u32)
        n4634 = Boolean Array To Number(Boolean array=w7056) -> (number=w7055:u32)
        n4635 = Boolean Array To Number(Boolean array=w7005) -> (number=w7004:u32)
        n4636 = Boolean Array To Number(Boolean array=w7029) -> (number=w7028:u32)
        n4637 = Boolean Array To Number(Boolean array=w7008) -> (number=w7009:u32)
        n4638 = Mantissa & Exponent(0:w7049) -> (2:w7050:dbl)  [unwired: 1 out]
        n4639 = Mantissa & Exponent(0:w7068) -> (2:w7069:dbl)  [unwired: 1 out]
        n4640 = Mantissa & Exponent(0:w7044) -> (2:w7047:dbl)  [unwired: 1 out]
        n4641 = Mantissa & Exponent(0:w7055) -> (2:w7054:dbl)  [unwired: 1 out]
        n4642 = Mantissa & Exponent(0:w7004) -> (2:w7003:dbl)  [unwired: 1 out]
        n4643 = Mantissa & Exponent(0:w7028) -> (2:w7027:dbl)  [unwired: 1 out]
        n4644 = Mantissa & Exponent(0:w7009) -> (2:w7010:dbl)  [unwired: 1 out]
        n4645 = case shown="1" w7069 {
          tunnel: [u32[][] [] ("data (RGB format)") w7089 w7090 w7091] -> w7070
          tunnel: w7065 -> [_ w7089 _ _]
          tunnel: w7064 -> [_ _ w7090 _]
          tunnel: w7063 -> [_ _ _ w7091]
          frame #0 {
          }
          frame #1 {
          }
          frame #2 {
          }
          frame #3 {
          }
        }
        n4646 = case shown="0, Default" w7047 {
          tunnel: [u32[][] [] ("data (RGB format)") w7086 w7087] -> w7046
          tunnel: w7043 -> [_ w7086 _]
          tunnel: w7042 -> [_ _ w7087]
          frame #0 {
          }
          frame #1 {
          }
          frame #2 {
          }
        }
        n4647 = case shown="0, Default" w7050 {
          tunnel: [u32[][] [] ("data (RGB format)") w7084] -> w7052
          tunnel: w7040 -> [_ w7084]
          frame #0 {
          }
          frame #1 {
          }
        }
        n4648 = case shown="1" w7054 {
          tunnel: w7038 -> [_ w7081 _]
          tunnel: [u32[][] [] ("data (RGB format)") w7081 w7082] -> w7053
          tunnel: w7039 -> [_ _ w7082]
          frame #0 {
          }
          frame #1 {
          }
          frame #2 {
          }
        }
        n4649 = case shown="1" w7003 {
          tunnel: w6999 -> [_ w7072 _]
          tunnel: [u32[][] [] ("data (RGB format)") w7072 w7073] -> w6992
          tunnel: w6994 -> [_ _ w7073]
          frame #0 {
          }
          frame #1 {
          }
          frame #2 {
          }
        }
        n4650 = case shown="2" w7027 {
          tunnel: w7023 -> [_ w7078 _]
          tunnel: [u32[][] [] ("data (RGB format)") w7078 w7079] -> w7020
          tunnel: w7022 -> [_ _ w7079]
          frame #0 {
          }
          frame #1 {
          }
          frame #2 {
          }
        }
        n4651 = case shown="2" w7010 {
          tunnel: w7007 -> [_ w7075 _]
          tunnel: [u32[][] [] ("data (RGB format)") w7075 w7076] -> w6993
          tunnel: w7006 -> [_ _ w7076]
          frame #0 {
          }
          frame #1 {
          }
          frame #2 {
          }
        }
        n4652 = call-poly <vilib>:"Draw Unflattened Pixmap.vi"("top left point(0, 0)"=cluster{"x":i16, "y":i16} {"x"=93, "y"=169}, "data (RGB format)"=w7066) -> ("new picture"=w7058:picture)  [unwired: 7 in]
        n4653 = call-poly <vilib>:"Draw Unflattened Pixmap.vi"("picture"=w7058, "top left point(0, 0)"=cluster{"x":i16, "y":i16} {"x"=182, "y"=297}, "data (RGB format)"=w7070) -> ("new picture"=w7041:picture)  [unwired: 6 in]
        n4654 = call-poly <vilib>:"Draw Unflattened Pixmap.vi"("picture"=w7041, "top left point(0, 0)"=cluster{"x":i16, "y":i16} {"x"=564, "y"=310}, "data (RGB format)"=w7046) -> ("new picture"=w7051:picture)  [unwired: 6 in]
        n4655 = call-poly <vilib>:"Draw Unflattened Pixmap.vi"("picture"=w7051, "top left point(0, 0)"=cluster{"x":i16, "y":i16} {"x"=282, "y"=593}, "data (RGB format)"=w7052) -> ("new picture"=w7057:picture)  [unwired: 6 in]
        n4656 = call-poly <vilib>:"Draw Unflattened Pixmap.vi"("picture"=w7057, "top left point(0, 0)"=cluster{"x":i16, "y":i16} {"x"=304, "y"=649}, "data (RGB format)"=w7053) -> ("new picture"=w7021:picture)  [unwired: 6 in]
        n4657 = call-poly <vilib>:"Draw Unflattened Pixmap.vi"("picture"=w7021, "top left point(0, 0)"=cluster{"x":i16, "y":i16} {"x"=92, "y"=313}, "data (RGB format)"=w7020) -> ("new picture"=w6998:picture)  [unwired: 6 in]
        n4658 = call-poly <vilib>:"Draw Unflattened Pixmap.vi"("picture"=w6998, "top left point(0, 0)"=cluster{"x":i16, "y":i16} {"x"=175, "y"=251}, "data (RGB format)"=w6993) -> ("new picture"=w6997:picture)  [unwired: 6 in]
        n4659 = call-poly <vilib>:"Draw Unflattened Pixmap.vi"("picture"=w6997, "top left point(0, 0)"=cluster{"x":i16, "y":i16} {"x"=488, "y"=250} ("top left point(0, 0) 2"), "data (RGB format)"=w6992) -> ("new picture"=w6996:picture)  [unwired: 6 in]
      }
      frame #1 {
        # "8"
        # "PET COOL"
        # "7"
        # "CST FIX"
        # "6"
        # "CST FIX"
        # "5"
        # "MAGNETRON"
        n4660 = property on="new picture 3" class="Pict"() -> ("Mouse"=w7173:T37)  [unwired: 2 in, 2 out]
        n4661 = Unbundle(w7173) -> ("Mouse Position"=w7172:cluster{"X":i32, "Y":i32}, "Mouse Modifiers"=w7180:T38)
        "Mouse Position 4" <- w7172
        n4662 = Unbundle(w7180) -> ("Button Down"=w7130:bool)  [unwired: 3 out]
        n4663 = Unbundle(w7172) -> ("X"=w7098:i32, "Y"=w7099:i32)
        n4664 = In Range and Coerce(upper limit=605, x=w7099, lower limit=324) -> (In Range?=w7159:bool)  [unwired: 1 out]
        n4665 = In Range and Coerce(upper limit=140, x=w7098, lower limit=98) -> (In Range?=w7158:bool)  [unwired: 1 out]
        n4666 = In Range and Coerce(upper limit=600, x=w7099, lower limit=324) -> (In Range?=w7174:bool)  [unwired: 1 out]
        n4667 = In Range and Coerce(upper limit=610, x=w7098, lower limit=570) -> (In Range?=w7175:bool)  [unwired: 1 out]
        n4668 = In Range and Coerce(upper limit=277, x=w7099, lower limit=252) -> (In Range?=w7149:bool)  [unwired: 1 out]
        n4669 = In Range and Coerce(upper limit=527, x=w7098, lower limit=490) -> (In Range?=w7150:bool)  [unwired: 1 out]
        n4670 = In Range and Coerce(upper limit=333, x=w7099, lower limit=171) -> (In Range?=w7105:bool)  [unwired: 1 out]
        n4671 = In Range and Coerce(upper limit=382, x=w7098, lower limit=327) -> (In Range?=w7104:bool)  [unwired: 1 out]
        n4672 = In Range and Coerce(upper limit=325, x=w7099, lower limit=203) -> (In Range?=w7106:bool)  [unwired: 1 out]
        n4673 = In Range and Coerce(upper limit=474, x=w7098, lower limit=435) -> (In Range?=w7107:bool)  [unwired: 1 out]
        n4674 = In Range and Coerce(upper limit=281, x=w7099, lower limit=256) -> (In Range?=w7148:bool)  [unwired: 1 out]
        n4675 = In Range and Coerce(upper limit=210, x=w7098, lower limit=185) -> (In Range?=w7147:bool)  [unwired: 1 out]
        n4676 = In Range and Coerce(upper limit=325, x=w7099, lower limit=203) -> (In Range?=w7117:bool)  [unwired: 1 out]
        n4677 = In Range and Coerce(upper limit=275, x=w7098, lower limit=235) -> (In Range?=w7116:bool)  [unwired: 1 out]
        n4678 = In Range and Coerce(upper limit=685, x=w7099, lower limit=641) -> (In Range?=w7137:bool)  [unwired: 1 out]
        n4679 = In Range and Coerce(upper limit=418, x=w7098, lower limit=283) -> (In Range?=w7138:bool)  [unwired: 1 out]
        n4680 = And(x=w7158, y=w7159) -> (x .and. y?=w7134:bool)
        n4681 = And(x=w7175, y=w7174) -> (x .and. y?=w7161:bool)
        n4682 = And(x=w7150, y=w7149) -> (x .and. y?=w7133:bool)
        n4683 = And(x=w7104, y=w7105) -> (x .and. y?=w7094:bool)
        n4684 = And(x=w7107, y=w7106) -> (x .and. y?=w7095:bool)
        n4685 = And(x=w7147, y=w7148) -> (x .and. y?=w7129:bool)
        n4686 = And(x=w7116, y=w7117) -> (x .and. y?=w7096:bool)
        n4687 = And(x=w7138, y=w7137) -> (x .and. y?=w7097:bool)
        n4688 = And(x=w7130, y=w7161) -> (x .and. y?=w7171:bool)
        n4689 = And(x=w7130, y=w7134) -> (x .and. y?=w7135:bool)
        n4690 = And(x=w7130, y=w7133) -> (x .and. y?=w7132:bool)
        n4691 = And(x=w7130, y=w7129) -> (x .and. y?=w7131:bool)
        n4692 = case shown="True" w7132 {
          frame #0 {
          }
          frame #1 {
            "Ch3_trns_gv_bp_timer_front" <- TRUE ("ch2_bv_R_timer_front")
          }
        }
        n4693 = case shown="True" w7171 {
          frame #0 {
          }
          frame #1 {
            "Gv_timer_front_ch3_2" <- TRUE ("Gv_timer_front_ch2_3")
          }
        }
        n4694 = case shown="True" w7135 {
          frame #0 {
          }
          frame #1 {
            "Gv_timer_front_ch3_4" <- TRUE ("Gv_timer_front_ch2_1")
          }
        }
        n4695 = case shown="True" w7131 {
          frame #0 {
          }
          frame #1 {
            "Ch3_trns_gv_bp2_timer_front" <- TRUE ("ch2_bv_L_timerl_front")
          }
        }
        n4696 = local read "Ch3_trns_gv_bp2_timer_front"() -> (w7093:bool)
        n4697 = local read "Ch3_trns_gv_bp_timer_front"() -> (w7092:bool)
        n4698 = Build Array(TRUE, w7161, w7134, w7133, w7129, w7097, w7096, w7095, w7094) -> (w7170:bool[])
        n4699 = local read "Gv_timer_front_ch3_4"() -> (w7118:bool)
        n4700 = local read "Gv_timer_front_ch3_2"() -> (w7119:bool)
        n4701 = Boolean Array To Number(Boolean array=w7170) -> (number=w7169:u32)
        n4702 = Mantissa & Exponent(0:w7169) -> (2:w7160:dbl)  [unwired: 1 out]
        n4703 = feedback #129() -> (w7124:bool)  [unwired: 1 in]
        n4704 = feedback #130() -> (w7123:bool)  [unwired: 1 in]
        n4705 = feedback #131() -> (w7126:bool)  [unwired: 1 in]